vi "UHR-Fleezers Control (host) - Avogadro v3.vi"() -> ()   [LabVIEW 2014] (continued)
                                frame #1 {
                                n2744 = Wait (ms)(milliseconds to wait=u32 500) -> ()  [unwired: 1 out]
                                }
                                frame #2 {
                                n2745 = local read "Shift confocal"() -> (w4245:bool)
                                n2746 = local read "Mean"() -> (w4247:dbl)
                                n2747 = Greater?(x=w4247, y=11.0) -> (0:w4244:bool)
                                n2748 = Not(x=w4244) -> (.not. x?=w4243:bool)
                                n2749 = And(x=w4243, y=w4245) -> (x .and. y?=w4241:bool)
                                n2750 = And(x=w4244, y=w4245) -> (x .and. y?=w4242:bool)
                                n2751 = case shown="True" w4242 {
                                frame False {
                                }
                                frame True {
                                n2752 = local read "Confocal Y 2 (V)"() -> (w4251:dbl)
                                n2753 = local read "Confocal X 2 (V)"() -> (w4250:dbl)
                                n2754 = property on="AO2" class="Slide (strict)"("Val(Sgnl)"=w4250) -> ()  [unwired: 2 in, 2 out]
                                n2755 = property on="AO1" class="Slide (strict)"("Val(Sgnl)"=w4251) -> ()  [unwired: 2 in, 2 out]
                                }
                                }
                                n2756 = case shown="True" w4241 {
                                frame False {
                                }
                                frame True {
                                n2757 = local read "Confocal X 1 (V)"() -> (w4248:dbl)
                                n2758 = local read "Confocal Y 1 (V)"() -> (w4249:dbl)
                                n2759 = property on="AO2" class="Slide (strict)"("Val(Sgnl)"=w4248) -> ()  [unwired: 2 in, 2 out]
                                n2760 = property on="AO1" class="Slide (strict)"("Val(Sgnl)"=w4249) -> ()  [unwired: 2 in, 2 out]
                                }
                                }
                                }
                                }
                                }
                                }
                                }
                                }
                                }
                                frame "Image" {
                                n2761 = property on="Confocal Image" class="Bool (strict)"("Val(Sgnl)"=TRUE ("Value (Signaling)")) -> ()  [unwired: 2 in, 2 out]
                                }
                              }
                              n2762 = local write "Fl. High"(FALSE ("Fl. High")) -> ()
                              n2763 = local read "Time (s)"() -> (w4185:dbl)
                            }
                            frame #1 {
                              n2764 = case shown="True" "Auto F Reset" {
                                tunnel: w4257 -> [_ w4262]
                                tunnel: w4256 -> [_ w4261]
                                tunnel: w4255 -> [_ w4260]
                                tunnel: w4254 -> [_ w4259]
                                frame False {
                                }
                                frame True {
                                n2765 = node-c288() -> (w4264:T43)  [unwired: 4 in]
                                n2766 = timed-loop {
                                timing: w4264 -> [_]
                                timing-out: [_] -> w4263
                                tunnel: w4262 -> [w4269]
                                tunnel: w4261 -> [w4268]
                                tunnel: w4260 -> [w4267]
                                tunnel: w4259 -> [w4266]
                                stop <- w4265 stop-if-true
                                n2767 = node-c288() -> ()  [unwired: 1 in, 1 out]
                                n2768 = local read "Fl. Delta Thresh. (kHz)"() -> (w4278:dbl)
                                n2769 = local read "APD to Watch"() -> (w4279:bool)
                                n2770 = local read "Delta Fl. 1"() -> (w4280:dbl)
                                n2771 = local read "Delta Fl. 2"() -> (w4281:dbl)
                                n2772 = local read "Fl. Triggered..."() -> (w4272:bool)
                                n2773 = local read "Stop All"() -> (w4273:bool)
                                n2774 = local read "Reset Force"() -> (w4271:bool)
                                n2775 = Multiply(x=w4278, y=1000.0) -> (x*y=w4276:dbl)
                                n2776 = Select(t=w4280, s=w4279, f=w4281) -> (s? t:f=w4275:dbl)
                                n2777 = Not(x=w4272) -> (.not. x?=w4270:bool)
                                n2778 = Greater?(x=w4275, y=w4276) -> (0:w4274:bool)
                                n2779 = Compound Arithmetic op=OR(w4274, w4273, w4270, w4271) -> (w4265:bool)
                                n2780 = case shown="True" w4265 {
                                tunnel: w4269 -> [_ w4285]
                                tunnel: w4268 -> [_ w4289]
                                tunnel: w4267 -> [_ w4288]
                                tunnel: w4266 -> [_ w4287]
                                frame False {
                                }
                                frame True {
                                n2781 = case shown="\"Yank\"" w4289 {
                                tunnel: w4288 -> [_ w4299]
                                tunnel: w4287 -> [_ w4297]
                                frame "Image", Default {
                                }
                                frame "Yank" {
                                n2782 = flat-sequence {
                                tunnel: [w4302] -> w4300
                                tunnel: w4299 -> [w4302]
                                tunnel: [w4301] -> w4298
                                tunnel: w4297 -> [w4301]
                                tunnel: w4300 -> [w4308]
                                tunnel: w4298 -> [w4306]
                                frame #0 {
                                n2783 = local read "Yank Delay (s)"() -> (w4305:dbl)
                                n2784 = Multiply(x=w4305, y=1000.0) -> (x*y=w4303:dbl)
                                n2785 = Wait (ms)(milliseconds to wait=w4303) -> ()  [unwired: 1 out]
                                }
                                frame #1 {
                                n2786 = local read "Yank to which?"() -> (w4307:bool)
                                n2787 = case shown="False" w4307 {
                                tunnel: w4308 -> [_ w4336]
                                tunnel: w4306 -> [w4309 _]
                                frame False {
                                n2788 = flat-sequence {
                                tunnel: w4309 -> [w4310]
                                frame #0 {
                                n2789 = property on="Trap Pos FB SP" class="DigNum (strict)"("Val(Sgnl)"=w4310) -> ()  [unwired: 2 in, 2 out]
                                }
                                frame #1 {
                                n2790 = Wait (ms)(milliseconds to wait=u32 700) -> ()  [unwired: 1 out]
                                }
                                frame #2 {
                                n2791 = local read "Action (%)"() -> (w4315:dbl)
                                n2792 = Absolute Value(x=w4315) -> (abs(x)=w4314:dbl)
                                n2793 = Greater?(x=w4314, y=70.0) -> (0:w4312:bool)
                                n2794 = property on="Remove Action Offset" class="Bool (strict)"("Val(Sgnl)"=w4312) -> ()  [unwired: 2 in, 2 out]
                                }
                                frame #3 {
                                n2795 = for {
                                N: 4 -> [_]
                                n2796 = flat-sequence {
                                frame #0 {
                                n2797 = Wait (ms)(milliseconds to wait=u32 500) -> ()  [unwired: 1 out]
                                }
                                frame #1 {
                                n2798 = local read "Action (%)"() -> (w4321:dbl)
                                n2799 = Absolute Value(x=w4321) -> (abs(x)=w4320:dbl)
                                n2800 = Greater?(x=w4320, y=70.0) -> (0:w4318:bool)
                                n2801 = property on="Remove Action Offset" class="Bool (strict)"("Val(Sgnl)"=w4318) -> ()  [unwired: 2 in, 2 out]
                                }
                                }
                                }
                                }
                                frame #4 {
                                n2802 = Wait (ms)(milliseconds to wait=u32 500) -> ()  [unwired: 1 out]
                                }
                                frame #5 {
                                n2803 = local read "Shift confocal"() -> (w4326:bool)
                                n2804 = local read "Mean"() -> (w4329:dbl)
                                n2805 = Greater?(x=w4329, y=11.0) -> (0:w4325:bool)
                                n2806 = Not(x=w4325) -> (.not. x?=w4324:bool)
                                n2807 = And(x=w4325, y=w4326) -> (x .and. y?=w4327:bool)
                                n2808 = And(x=w4324, y=w4326) -> (x .and. y?=w4323:bool)
                                n2809 = case shown="True" w4327 {
                                frame False {
                                }
                                frame True {
                                n2810 = local read "Confocal X 2 (V)"() -> (w4332:dbl)
                                n2811 = local read "Confocal Y 2 (V)"() -> (w4333:dbl)
                                n2812 = property on="AO2" class="Slide (strict)"("Val(Sgnl)"=w4332) -> ()  [unwired: 2 in, 2 out]
                                n2813 = property on="AO1" class="Slide (strict)"("Val(Sgnl)"=w4333) -> ()  [unwired: 2 in, 2 out]
                                }
                                }
                                n2814 = case shown="True" w4323 {
                                frame False {
                                }
                                frame True {
                                n2815 = local read "Confocal Y 1 (V)"() -> (w4331:dbl)
                                n2816 = local read "Confocal X 1 (V)"() -> (w4330:dbl)
                                n2817 = property on="AO1" class="Slide (strict)"("Val(Sgnl)"=w4331) -> ()  [unwired: 2 in, 2 out]
                                n2818 = property on="AO2" class="Slide (strict)"("Val(Sgnl)"=w4330) -> ()  [unwired: 2 in, 2 out]
                                }
                                }
                                }
                                frame #6 {
                                n2819 = Wait (ms)(milliseconds to wait=u32 1500) -> ()  [unwired: 1 out]
                                }
                                frame #7 {
                                n2820 = property on="Rem fb disp offset" class="Bool (strict)"("Val(Sgnl)"=TRUE ("Value (Signaling)")) -> ()  [unwired: 2 in, 2 out]
                                }
                                }
                                }
                                frame True {
                                n2821 = flat-sequence {
                                tunnel: w4336 -> [w4337]
                                frame #0 {
                                n2822 = property on="Trap Delta (MHz)" class="DigNum (strict)"("Val(Sgnl)"=w4337) -> ()  [unwired: 2 in, 2 out]
                                }
                                frame #1 {
                                n2823 = Wait (ms)(milliseconds to wait=u32 500) -> ()  [unwired: 1 out]
                                }
                                frame #2 {
                                n2824 = local read "Shift confocal"() -> (w4343:bool)
                                n2825 = local read "Mean"() -> (w4344:dbl)
                                n2826 = Greater?(x=w4344, y=11.0) -> (0:w4342:bool)
                                n2827 = And(x=w4342, y=w4343) -> (x .and. y?=w4340:bool)
                                n2828 = Not(x=w4342) -> (.not. x?=w4341:bool)
                                n2829 = And(x=w4341, y=w4343) -> (x .and. y?=w4339:bool)
                                n2830 = case shown="True" w4340 {
                                frame False {
                                }
                                frame True {
                                n2831 = local read "Confocal Y 2 (V)"() -> (w4349:dbl)
                                n2832 = local read "Confocal X 2 (V)"() -> (w4348:dbl)
                                n2833 = property on="AO1" class="Slide (strict)"("Val(Sgnl)"=w4349) -> ()  [unwired: 2 in, 2 out]
                                n2834 = property on="AO2" class="Slide (strict)"("Val(Sgnl)"=w4348) -> ()  [unwired: 2 in, 2 out]
                                }
                                }
                                n2835 = case shown="True" w4339 {
                                frame False {
                                }
                                frame True {
                                n2836 = local read "Confocal Y 1 (V)"() -> (w4347:dbl)
                                n2837 = local read "Confocal X 1 (V)"() -> (w4346:dbl)
                                n2838 = property on="AO2" class="Slide (strict)"("Val(Sgnl)"=w4346) -> ()  [unwired: 2 in, 2 out]
                                n2839 = property on="AO1" class="Slide (strict)"("Val(Sgnl)"=w4347) -> ()  [unwired: 2 in, 2 out]
                                }
                                }
                                }
                                }
                                }
                                }
                                }
                                }
                                }
                                }
                                n2840 = local read "Time (s)"() -> (w4284:dbl)
                                n2841 = Subtract(x=w4285, y=w4284) -> (x-y=w4296:dbl)
                                n2842 = Number To Decimal String(number=w4296, width (-)=i16 0) -> (decimal integer string=w4294:string)
                                n2843 = Concatenate Strings(w4294, " s fluorescence event") -> (w4291:string)
                                n2844 = local read "Messages"() -> (w4292:string)
                                n2845 = local write "Duration (s)"(w4296) -> ()
                                n2846 = call "Update messages.vi"("Message to add"=w4291, "Old message string"=w4292) -> ("New message string"=w4290:string)
                                n2847 = local write "Messages"(w4290) -> ()
                                n2848 = call <vilib>:"Beep.vi"() -> ()  [unwired: 12 in]
                                n2849 = local write "Reset Force"(FALSE ("Force Reset")) -> ()
                                n2850 = local write "Fl. High"(TRUE ("Fl. High")) -> ()
                                n2851 = local write "Waiting"(TRUE ("Waiting")) -> ()
                                }
                                }
                                n2852 = node-c288() -> ()  [unwired: 1 in, 1 out]
                                }
                                n2853 = node-c288(w4263) -> ()  [unwired: 1 out]
                                }
                              }
                            }
                          }
                          n2854 = local read "Trap Delta (MHz)"() -> (w4175:dbl)
                          n2855 = local read "Trap Pos FB SP"() -> (w4173:fxp<+/-,16,1>)
                        }
                      }
                    }
                    frame True {
                      n2856 = flat-sequence {
                        tunnel: w4360 -> [w4370]
                        tunnel: [w4370] -> w4364
                        tunnel: w4363 -> [w4369]
                        tunnel: [w4369] -> w4362
                        tunnel: [w4368] -> w4361
                        tunnel: w4359 -> [w4367]
                        tunnel: [w4366] -> w4358
                        tunnel: w4355 -> [w4365]
                        tunnel: [w4365] -> w4354
                        tunnel: w4364 -> [w4440]
                        tunnel: w4362 -> [w4439]
                        tunnel: w4361 -> [w4438]
                        tunnel: w4358 -> [w4437]
                        tunnel: w4354 -> [w4436]
                        tunnel: [w4437] -> w4357
                        frame #0 {
                          n2857 = call <vilib>:"Beep.vi"() -> ()  [unwired: 3 in, 9 out]
                          n2858 = local write "Waiting"(FALSE ("Waiting")) -> ()
                          n2859 = Increment(x=w4367) -> (x+1=w4366:u8)
                          n2860 = case shown="\"Image\"" w4369 {
                            tunnel: w4366 -> [_ _ w4376]
                            frame "Image" {
                              n2861 = property on="Confocal Image" class="Bool (strict)"("Val(Sgnl)"=TRUE ("Value (Signaling)")) -> ()  [unwired: 2 in, 2 out]
                            }
                            frame "Alarm", Default {
                            }
                            frame "Yank" {
                              n2862 = flat-sequence {
                                tunnel: w4376 -> [w4379]
                                tunnel: [w4378] -> w4375
                                tunnel: ["N Array El"] -> w4374
                                tunnel: w4375 -> [w4393]
                                tunnel: w4374 -> [w4389]
                                frame #0 {
                                n2863 = Multiply(x="Yank Delay (s)", y=1000.0) -> (x*y=w4382:dbl)
                                n2864 = Quotient & Remainder(x=w4379, y="N Array El") -> (x-y*floor(x/y)=w4378:u8)  [unwired: 1 out]
                                n2865 = Wait (ms)(milliseconds to wait=w4382) -> ()  [unwired: 1 out]
                                }
                                frame #1 {
                                n2866 = Random Number (0-1)() -> (number: 0 to 1=w4390:dbl)
                                n2867 = Multiply(x=w4389, y=w4390) -> (x*y=w4388:dbl)
                                n2868 = Round Toward -Infinity(1:w4388) -> (0:w4387:dbl)
                                n2869 = Select(t=w4387, s="Random Choice", f=w4393) -> (s? t:f=w4391:dbl)
                                n2870 = Select(t="Yank to Trap Delta (MHz)", s="Yank to which?", f="Yank to SP") -> (s? t:f=w4384:dbl[])
                                n2871 = Index Array(array=w4384, index=w4391) -> (element=w4394:dbl)
                                n2872 = case shown="False" "Yank to which?" {
                                tunnel: w4394 -> [w4395 w4421]
                                frame False {
                                n2873 = flat-sequence {
                                tunnel: w4395 -> [w4396]
                                frame #0 {
                                n2874 = property on="Trap Pos FB SP" class="DigNum (strict)"("Val(Sgnl)"=w4396) -> ()  [unwired: 2 in, 2 out]
                                }
                                frame #1 {
                                n2875 = Wait (ms)(milliseconds to wait=u32 700) -> ()  [unwired: 1 out]
                                }
                                frame #2 {
                                n2876 = local read "Action (%)"() -> (w4401:dbl)
                                n2877 = Absolute Value(x=w4401) -> (abs(x)=w4400:dbl)
                                n2878 = Greater?(x=w4400, y=70.0) -> (0:w4398:bool)
                                n2879 = property on="Remove Action Offset" class="Bool (strict)"("Val(Sgnl)"=w4398) -> ()  [unwired: 2 in, 2 out]
                                }
                                frame #3 {
                                n2880 = for {
                                N: 4 -> [_]
                                n2881 = flat-sequence {
                                frame #0 {
                                n2882 = Wait (ms)(milliseconds to wait=u32 500) -> ()  [unwired: 1 out]
                                }
                                frame #1 {
                                n2883 = local read "Action (%)"() -> (w4407:dbl)
                                n2884 = Absolute Value(x=w4407) -> (abs(x)=w4406:dbl)
                                n2885 = Greater?(x=w4406, y=70.0) -> (0:w4404:bool)
                                n2886 = property on="Remove Action Offset" class="Bool (strict)"("Val(Sgnl)"=w4404) -> ()  [unwired: 2 in, 2 out]
                                }
                                }
                                }
                                }
                                frame #4 {
                                n2887 = local read "Shift confocal"() -> (w4411:bool)
                                n2888 = local read "Mean"() -> (w4414:dbl)
                                n2889 = Greater?(x=w4414, y=11.0) -> (0:w4410:bool)
                                n2890 = Not(x=w4410) -> (.not. x?=w4409:bool)
                                n2891 = And(x=w4409, y=w4411) -> (x .and. y?=w4408:bool)
                                n2892 = And(x=w4410, y=w4411) -> (x .and. y?=w4412:bool)
                                n2893 = case shown="True" w4412 {
                                frame False {
                                }
                                frame True {
                                n2894 = local read "Confocal X 2 (V)"() -> (w4417:dbl)
                                n2895 = local read "Confocal Y 2 (V)"() -> (w4418:dbl)
                                n2896 = property on="AO2" class="Slide (strict)"("Val(Sgnl)"=w4417) -> ()  [unwired: 2 in, 2 out]
                                n2897 = property on="AO1" class="Slide (strict)"("Val(Sgnl)"=w4418) -> ()  [unwired: 2 in, 2 out]
                                }
                                }
                                n2898 = case shown="True" w4408 {
                                frame False {
                                }
                                frame True {
                                n2899 = local read "Confocal X 1 (V)"() -> (w4415:dbl)
                                n2900 = local read "Confocal Y 1 (V)"() -> (w4416:dbl)
                                n2901 = property on="AO1" class="Slide (strict)"("Val(Sgnl)"=w4416) -> ()  [unwired: 2 in, 2 out]
                                n2902 = property on="AO2" class="Slide (strict)"("Val(Sgnl)"=w4415) -> ()  [unwired: 2 in, 2 out]
                                }
                                }
                                }
                                frame #5 {
                                n2903 = Wait (ms)(milliseconds to wait=u32 1500) -> ()  [unwired: 1 out]
                                }
                                frame #6 {
                                n2904 = property on="Rem fb disp offset" class="Bool (strict)"("Val(Sgnl)"=TRUE ("Value (Signaling)")) -> ()  [unwired: 2 in, 2 out]
                                }
                                }
                                }
                                frame True {
                                n2905 = flat-sequence {
                                tunnel: w4421 -> [w4422]
                                frame #0 {
                                n2906 = property on="Trap Delta (MHz)" class="DigNum (strict)"("Val(Sgnl)"=w4422) -> ()  [unwired: 2 in, 2 out]
                                }
                                frame #1 {
                                n2907 = Wait (ms)(milliseconds to wait=u32 500) -> ()  [unwired: 1 out]
                                }
                                frame #2 {
                                n2908 = local read "Shift confocal"() -> (w4426:bool)
                                n2909 = local read "Mean"() -> (w4424:dbl)
                                n2910 = Greater?(x=w4424, y=11.0) -> (0:w4427:bool)
                                n2911 = Not(x=w4427) -> (.not. x?=w4428:bool)
                                n2912 = And(x=w4428, y=w4426) -> (x .and. y?=w4430:bool)
                                n2913 = And(x=w4427, y=w4426) -> (x .and. y?=w4429:bool)
                                n2914 = case shown="True" w4429 {
                                frame False {
                                }
                                frame True {
                                n2915 = local read "Confocal Y 2 (V)"() -> (w4434:dbl)
                                n2916 = local read "Confocal X 2 (V)"() -> (w4433:dbl)
                                n2917 = property on="AO1" class="Slide (strict)"("Val(Sgnl)"=w4434) -> ()  [unwired: 2 in, 2 out]
                                n2918 = property on="AO2" class="Slide (strict)"("Val(Sgnl)"=w4433) -> ()  [unwired: 2 in, 2 out]
                                }
                                }
                                n2919 = case shown="True" w4430 {
                                frame False {
                                }
                                frame True {
                                n2920 = local read "Confocal X 1 (V)"() -> (w4431:dbl)
                                n2921 = local read "Confocal Y 1 (V)"() -> (w4432:dbl)
                                n2922 = property on="AO2" class="Slide (strict)"("Val(Sgnl)"=w4431) -> ()  [unwired: 2 in, 2 out]
                                n2923 = property on="AO1" class="Slide (strict)"("Val(Sgnl)"=w4432) -> ()  [unwired: 2 in, 2 out]
                                }
                                }
                                }
                                }
                                }
                                }
                                }
                              }
                            }
                          }
                          n2924 = local read "Time (s)"() -> (w4368:dbl)
                          "Fl. High" <- TRUE ("Yanking")
                        }
                        frame #1 {
                          n2925 = local read "Auto F Reset"() -> (w4435:bool)
                          n2926 = case shown="True" w4435 {
                            tunnel: w4440 -> [_ w4444]
                            tunnel: w4439 -> [_ w4443]
                            tunnel: w4438 -> [_ w4442]
                            tunnel: w4436 -> [_ w4441]
                            frame False {
                            }
                            frame True {
                              n2927 = node-c288() -> (w4446:T43)  [unwired: 4 out]
                              n2928 = timed-loop {
                                timing: w4446 -> [_]
                                timing-out: [_] -> w4445
                                tunnel: w4444 -> [w4464]
                                tunnel: w4443 -> [w4463]
                                tunnel: w4442 -> [w4462]
                                tunnel: w4441 -> [w4461]
                                stop <- w4447 stop-if-true
                                n2929 = node-c288() -> ()  [unwired: 2 out]
                                n2930 = local read "Fl. Delta Thresh. (kHz)"() -> (w4455:dbl)
                                n2931 = local read "Fl. Triggered..."() -> (w4460:bool)
                                n2932 = local read "Delta Fl. 1"() -> (w4451:dbl)
                                n2933 = local read "Delta Fl. 2"() -> (w4449:dbl)
                                n2934 = local read "Stop All"() -> (w4458:bool)
                                n2935 = local read "APD to Watch"() -> (w4450:bool)
                                n2936 = Select(t=w4451, s=w4450, f=w4449) -> (s? t:f=w4448:dbl)
                                n2937 = Not(x=w4460) -> (.not. x?=w4459:bool)
                                n2938 = Multiply(x=w4455, y=1000.0) -> (x*y=w4454:dbl)
                                n2939 = Negate(x=w4454) -> (-x=w4453:dbl)
                                n2940 = Less?(x=w4448, y=w4453) -> (x < y?=w4457:bool)
                                n2941 = Compound Arithmetic op=OR(w4457, w4458, w4459, "Reset Force") -> (w4447:bool)
                                n2942 = case shown="True" w4447 {
                                tunnel: w4464 -> [_ w4479]
                                tunnel: w4463 -> [_ w4478]
                                tunnel: w4462 -> [_ w4468]
                                tunnel: w4461 -> [_ w4470]
                                frame False {
                                }
                                frame True {
                                n2943 = local read "Time (s)"() -> (w4469:dbl)
                                n2944 = case shown="\"Yank\"" w4478 {
                                tunnel: w4479 -> [_ w4482]
                                tunnel: w4470 -> [_ w4480]
                                frame "Image", Default {
                                }
                                frame "Yank" {
                                n2945 = flat-sequence {
                                tunnel: [w4488] -> w4483
                                tunnel: w4482 -> [w4488]
                                tunnel: [w4484] -> w4481
                                tunnel: w4480 -> [w4484]
                                tunnel: w4483 -> [w4491]
                                tunnel: w4481 -> [w4489]
                                frame #0 {
                                n2946 = local read "Yank Delay (s)"() -> (w4487:dbl)
                                n2947 = Multiply(x=w4487, y=1000.0) -> (x*y=w4485:dbl)
                                n2948 = Wait (ms)(milliseconds to wait=w4485) -> ()  [unwired: 1 out]
                                }
                                frame #1 {
                                n2949 = local read "Yank to which?"() -> (w4490:bool)
                                n2950 = case shown="False" w4490 {
                                tunnel: w4491 -> [_ w4518]
                                tunnel: w4489 -> [w4492 _]
                                frame False {
                                n2951 = flat-sequence {
                                tunnel: w4492 -> [w4493]
                                frame #0 {
                                n2952 = property on="Trap Pos FB SP" class="DigNum (strict)"("Val(Sgnl)"=w4493) -> ()  [unwired: 2 in, 2 out]
                                }
                                frame #1 {
                                n2953 = Wait (ms)(milliseconds to wait=u32 700) -> ()  [unwired: 1 out]
                                }
                                frame #2 {
                                n2954 = local read "Action (%)"() -> (w4498:dbl)
                                n2955 = Absolute Value(x=w4498) -> (abs(x)=w4497:dbl)
                                n2956 = Greater?(x=w4497, y=70.0) -> (0:w4495:bool)
                                n2957 = property on="Remove Action Offset" class="Bool (strict)"("Val(Sgnl)"=w4495) -> ()  [unwired: 2 in, 2 out]
                                }
                                frame #3 {
                                n2958 = for {
                                N: 4 -> [_]
                                n2959 = flat-sequence {
                                frame #0 {
                                n2960 = Wait (ms)(milliseconds to wait=u32 500) -> ()  [unwired: 1 out]
                                }
                                frame #1 {
                                n2961 = local read "Action (%)"() -> (w4504:dbl)
                                n2962 = Absolute Value(x=w4504) -> (abs(x)=w4503:dbl)
                                n2963 = Greater?(x=w4503, y=70.0) -> (0:w4501:bool)
                                n2964 = property on="Remove Action Offset" class="Bool (strict)"("Val(Sgnl)"=w4501) -> ()  [unwired: 2 in, 2 out]
                                }
                                }
                                }
                                }
                                frame #4 {
                                n2965 = local read "Shift confocal"() -> (w4509:bool)
                                n2966 = local read "Mean"() -> (w4511:dbl)
                                n2967 = Greater?(x=w4511, y=11.0) -> (0:w4508:bool)
                                n2968 = Not(x=w4508) -> (.not. x?=w4507:bool)
                                n2969 = And(x=w4508, y=w4509) -> (x .and. y?=w4506:bool)
                                n2970 = And(x=w4507, y=w4509) -> (x .and. y?=w4505:bool)
                                n2971 = case shown="True" w4506 {
                                frame False {
                                }
                                frame True {
                                n2972 = local read "Confocal Y 2 (V)"() -> (w4515:dbl)
                                n2973 = local read "Confocal X 2 (V)"() -> (w4514:dbl)
                                n2974 = property on="AO2" class="Slide (strict)"("Val(Sgnl)"=w4514) -> ()  [unwired: 2 in, 2 out]
                                n2975 = property on="AO1" class="Slide (strict)"("Val(Sgnl)"=w4515) -> ()  [unwired: 2 in, 2 out]
                                }
                                }
                                n2976 = case shown="True" w4505 {
                                frame False {
                                }
                                frame True {
                                n2977 = local read "Confocal X 1 (V)"() -> (w4512:dbl)
                                n2978 = local read "Confocal Y 1 (V)"() -> (w4513:dbl)
                                n2979 = property on="AO1" class="Slide (strict)"("Val(Sgnl)"=w4513) -> ()  [unwired: 2 in, 2 out]
                                n2980 = property on="AO2" class="Slide (strict)"("Val(Sgnl)"=w4512) -> ()  [unwired: 2 in, 2 out]
                                }
                                }
                                }
                                frame #5 {
                                n2981 = Wait (ms)(milliseconds to wait=u32 1500) -> ()  [unwired: 1 out]
                                }
                                frame #6 {
                                n2982 = property on="Rem fb disp offset" class="Bool (strict)"("Val(Sgnl)"=TRUE ("Value (Signaling)")) -> ()  [unwired: 2 in, 2 out]
                                }
                                }
                                }
                                frame True {
                                n2983 = flat-sequence {
                                tunnel: w4518 -> [w4519]
                                frame #0 {
                                n2984 = property on="Trap Delta (MHz)" class="DigNum (strict)"("Val(Sgnl)"=w4519) -> ()  [unwired: 2 in, 2 out]
                                }
                                frame #1 {
                                n2985 = Wait (ms)(milliseconds to wait=u32 500) -> ()  [unwired: 1 out]
                                }
                                frame #2 {
                                n2986 = local read "Shift confocal"() -> (w4525:bool)
                                n2987 = local read "Mean"() -> (w4527:dbl)
                                n2988 = Greater?(x=w4527, y=11.0) -> (0:w4524:bool)
                                n2989 = Not(x=w4524) -> (.not. x?=w4523:bool)
                                n2990 = And(x=w4524, y=w4525) -> (x .and. y?=w4522:bool)
                                n2991 = And(x=w4523, y=w4525) -> (x .and. y?=w4521:bool)
                                n2992 = case shown="True" w4522 {
                                frame False {
                                }
                                frame True {
                                n2993 = local read "Confocal Y 2 (V)"() -> (w4531:dbl)
                                n2994 = local read "Confocal X 2 (V)"() -> (w4530:dbl)
                                n2995 = property on="AO2" class="Slide (strict)"("Val(Sgnl)"=w4530) -> ()  [unwired: 2 in, 2 out]
                                n2996 = property on="AO1" class="Slide (strict)"("Val(Sgnl)"=w4531) -> ()  [unwired: 2 in, 2 out]
                                }
                                }
                                n2997 = case shown="True" w4521 {
                                frame False {
                                }
                                frame True {
                                n2998 = local read "Confocal Y 1 (V)"() -> (w4529:dbl)
                                n2999 = local read "Confocal X 1 (V)"() -> (w4528:dbl)
                                n3000 = property on="AO2" class="Slide (strict)"("Val(Sgnl)"=w4528) -> ()  [unwired: 2 in, 2 out]
                                n3001 = property on="AO1" class="Slide (strict)"("Val(Sgnl)"=w4529) -> ()  [unwired: 2 in, 2 out]
                                }
                                }
                                }
                                }
                                }
                                }
                                }
                                }
                                }
                                }
                                n3002 = local read "Messages"() -> (w4477:string)
                                n3003 = Subtract(x=w4469, y=w4468) -> (x-y=w4475:dbl)
                                "Duration (s)" <- w4475
                                n3004 = Number To Decimal String(number=w4475, width (-)=i16 0) -> (decimal integer string=w4473:string)
                                n3005 = Concatenate Strings(w4473, " s fluorescence event." ("string")) -> (w4471:string)
                                n3006 = call "Update messages.vi"("Message to add"=w4471, "Old message string"=w4477) -> ("New message string"=w4476:string)
                                n3007 = local write "Reset Force"(FALSE ("Reset Force")) -> ()
                                n3008 = local write "Waiting"(TRUE ("Waiting")) -> ()
                                n3009 = local write "Messages"(w4476) -> ()
                                n3010 = local write "Fl. High"(FALSE ("Fl. High")) -> ()
                                n3011 = call <vilib>:"Beep.vi"() -> ()  [unwired: 3 in, 9 out]
                                }
                                }
                                n3012 = node-c288() -> ()  [unwired: 2 out]
                              }
                              n3013 = node-c288(w4445) -> ()  [unwired: 1 out]
                            }
                          }
                        }
                      }
                      n3014 = local read "Trap Delta (MHz)"() -> (w4360:dbl)
                      n3015 = local read "Trap Pos FB SP"() -> (w4355:fxp<+/-,16,1>)
                    }
                  }
                }
                frame #1 {
                  n3016 = local read "Stop All"() -> (w4541:bool)
                  n3017 = local read "Fl. Triggered..."() -> (w4539:bool)
                  n3018 = Not(x=w4539) -> (.not. x?=w4540:bool)
                  n3019 = Or(x=w4540, y=w4541) -> (x .or. y?=w4538:bool)
                }
              }
              n3020 = case shown="True" w4132 {
                frame False {
                }
                frame True {
                  n3021 = local read "Confocal Y 1 (V)"() -> (w4142:dbl)
                  n3022 = local read "Confocal X 1 (V)"() -> (w4141:dbl)
                  n3023 = property on="AO2" class="Slide (strict)"("Val(Sgnl)"=w4141) -> ()  [unwired: 2 in, 2 out]
                  n3024 = property on="AO1" class="Slide (strict)"("Val(Sgnl)"=w4142) -> ()  [unwired: 2 in, 2 out]
                }
              }
              n3025 = case shown="True" w4132 {
                frame False {
                }
                frame True {
                  w4140 = FALSE ("Fl. High")
                  n3026 = local write "Waiting"(w4140) -> ()
                  n3027 = local write "Fl. High"(w4140) -> ()
                }
              }
              n3028 = node-c288() -> ()  [unwired: 2 out]
            }
            n3029 = node-c288(w4130) -> ()  [unwired: 1 out]
          }
        }
      }
      event "Start assembly line": Value Change {
        n3030 = event-data() -> ()  [unwired: 7 out]
        n3031 = case shown="True" "Start assembly line" {
          tunnel: w4547 -> [_ w4548]
          frame False {
          }
          frame True {
            n3032 = flat-sequence {
              tunnel: w4548 -> [w4553]
              tunnel: [w4552] -> w4550
              tunnel: w4550 -> [w4585]
              tunnel: [w4584] -> w4549
              tunnel: w4549 -> [w4587]
              tunnel: w4548 -> [w4606]
              frame #0 {
                w4551 = TRUE ("Value (Signaling)")
                n3033 = property on="Vortran Laser ON" class="Bool (strict)"("Val(Sgnl)"=w4551) -> ()  [unwired: 2 in, 2 out]
                "AL Running" <- w4551
              }
              frame #1 {
                n3034 = node-c288() -> (w4555:T43)  [unwired: 4 in]
                n3035 = timed-loop {
                  timing: w4555 -> [_]
                  timing-out: [_] -> w4554
                  tunnel: w4553 -> [w4563]
                  tunnel: [w4558] -> w4552
                  stop <- w4559 stop-if-true
                  n3036 = node-c288() -> ()  [unwired: 1 in, 1 out]
                  n3037 = local read "APD rates cluster"() -> (w4557:T2)
                  n3038 = Multiply(x="Cy3 Fl.  Thresh. (kHz)", y=1000.0) -> (x*y=w4566:dbl)
                  n3039 = Unbundle By Name(w4557) -> ("APD 1 Rate (Hz)"=w4556:dbl)
                  n3040 = Greater?(x=w4556, y=w4566) -> (0:w4562:bool)
                  n3041 = case shown="True" w4562 {
                    tunnel: w4563 -> [_ w4569]
                    tunnel: [TRUE ("Stage Moving") w4568] -> w4561
                    frame False {
                    }
                    frame True {
                      n3042 = flat-sequence {
                        tunnel: w4569 -> [w4574]
                        tunnel: [w4579] -> w4568
                        frame #0 {
                          n3043 = Multiply(x="AL Delay (s)", y=u32 1000) -> (x*y=w4571:u32)
                          n3044 = Wait (ms)(milliseconds to wait=w4571) -> ()  [unwired: 1 out]
                        }
                        frame #1 {
                          n3045 = property on="Vortran Laser ON" class="Bool (strict)"("Val(Sgnl)"=FALSE ("Value (Signaling)")) -> ()  [unwired: 2 in, 2 out]
                        }
                        frame #2 {
                          # "upper spot"
                          n3046 = local read "Saved Stage Positions"() -> (w4577:dbl[][])
                          n3047 = local write "Stage Moving"(TRUE ("Stage Moving")) -> ()
                          n3048 = call "move to saved stage position.vi"("Stage VISA resource name in"=w4574, "Position"=5, "Saved Stage Positions"=w4577) -> ("error out"=w4575:errorcluster)  [unwired: 1 in, 1 out]
                          n3049 = local write "Stage Control Serial Error"(w4575) -> ()
                        }
                        frame #3 {
                          w4579 = FALSE ("Stage Moving")
                          n3050 = call <vilib>:"Beep.vi"() -> ()  [unwired: 3 in, 9 out]
                          n3051 = local write "Stage Moving"(w4579) -> ()
                        }
                      }
                    }
                  }
                  n3052 = local read "Stop assembly line"() -> (w4558:bool)
                  n3053 = Not(x=w4561) -> (.not. x?=w4560:bool)
                  n3054 = node-c288() -> ()  [unwired: 1 in, 1 out]
                  n3055 = Or(x=w4560, y=w4558) -> (x .or. y?=w4559:bool)
                }
                n3056 = node-c288(w4554) -> ()  [unwired: 1 out]
              }
              frame #2 {
                n3057 = Not(x=w4585) -> (.not. x?=w4584:bool)
                n3058 = case shown="True" w4584 {
                  frame False {
                  }
                  frame True {
                    n3059 = property on="Red Laser ON" class="Bool (strict)"("Val(Sgnl)"=TRUE ("Value (Signaling)")) -> ()  [unwired: 2 in, 2 out]
                  }
                }
              }
              frame #3 {
                n3060 = node-c288() -> (w4589:T43)  [unwired: 4 in]
                n3061 = timed-loop {
                  timing: w4589 -> [_]
                  timing-out: [_] -> w4588
                  tunnel: [w4592] -> _
                  tunnel: w4587 -> [w4592]
                  stop <- "Stop assembly line" stop-if-true
                  n3062 = node-c288() -> ()  [unwired: 1 in, 1 out]
                  n3063 = local read "APD rates cluster"() -> (w4591:T2)
                  n3064 = Multiply(x="Cy5 Fl.  Thresh. (kHz)", y=1000.0) -> (x*y=w4598:dbl)
                  n3065 = Unbundle By Name(w4591) -> ("APD 2 Rate (Hz)"=w4590:dbl)
                  n3066 = Greater?(x=w4590, y=w4598) -> (0:w4595:bool)
                  n3067 = And(x=w4595, y=w4592) -> (x .and. y?=w4593:bool)
                  n3068 = case shown="True" w4593 {
                    frame False {
                    }
                    frame True {
                      n3069 = property on="Vortran Laser ON" class="Bool (strict)"("Val(Sgnl)"=TRUE ("Value (Signaling)")) -> ()  [unwired: 2 in, 2 out]
                    }
                  }
                  n3070 = node-c288() -> ()  [unwired: 1 in, 1 out]
                }
                n3071 = node-c288(w4588) -> ()  [unwired: 1 out]
              }
              frame #4 {
                w4605 = FALSE ("Value (Signaling)")
                # "lower spot"
                n3072 = local read "Saved Stage Positions"() -> (w4609:dbl[][])
                n3073 = property on="Red Laser ON" class="Bool (strict)"("Val(Sgnl)"=w4605) -> ()  [unwired: 2 in, 2 out]
                n3074 = property on="Vortran Laser ON" class="Bool (strict)"("Val(Sgnl)"=w4605) -> ()  [unwired: 2 in, 2 out]
                n3075 = local write "Stage Moving"(TRUE ("Stage Moving")) -> ()
                n3076 = local write "Stop assembly line"(FALSE ("Stop assembly line")) -> ()
                n3077 = call "move to saved stage position.vi"("Stage VISA resource name in"=w4606, "Position"=3, "Saved Stage Positions"=w4609) -> ("error out"=w4608:errorcluster)  [unwired: 1 in, 1 out]
                n3078 = local write "Stage Control Serial Error"(w4608) -> ()
              }
              frame #5 {
                w4611 = FALSE ("Stage Moving")
                n3079 = local write "Stage Moving"(w4611) -> ()
                n3080 = local write "AL Running"(w4611) -> ()
                n3081 = call <vilib>:"Beep.vi"() -> ()  [unwired: 3 in, 9 out]
              }
            }
          }
        }
      }
      event "Stop All": Value Change {
        n3082 = event-data() -> ()  [unwired: 7 out]
        n3083 = local read "Stop All"() -> (w4612:bool)
      }
    }
    n3084 = node-c288() -> ()  [unwired: 2 out]
  }
  n3085 = node-c288(w52) -> ()  [unwired: 1 out]
  n3086 = node-c288(w63) -> ()  [unwired: 1 out]
  n3087 = node-c288(w61) -> ()  [unwired: 1 out]
  n3088 = property on="Saved trap pos" class="WFGraph (strict)"("Visible"=FALSE) -> ()  [unwired: 2 in, 2 out]
  n3089 = property on="Trap Delta Graph" class="WFGraph (strict)"("Visible"=TRUE) -> ()  [unwired: 2 in, 2 out]
  n3090 = disable-structure shown="Disabled" {
    disable-tunnel: w55 -> [w4614 _]
    disable-tunnel: w54 -> [w4613 _]
    frame Disabled {
      n3091 = VISA Close(VISA resource name=w4614, error in (no error)=w4613) -> (error out=w4615:errorcluster)
      n3092 = call <vilib>:"Simple Error Handler.vi"("error in (no error)"=w4615) -> ()  [unwired: 1 in, 8 out]
    }
    frame Enabled {
    }
  }
  n3093 = disable-structure shown="Disabled" {
    disable-tunnel: [w4623 _] -> w20
    disable-tunnel: [w4619 _] -> w19
    disable-tunnel: [w4618 _] -> w18
    disable-tunnel: [w4617 _] -> w17
    disable-tunnel: [w4616 _] -> w16
    frame Disabled {
      # "n samples needed for data"
      n3094 = Unbundle By Name("sound format") -> ("sample rate (S/s)"=w4619:dbl)
      n3095 = call <vilib>:"Sound Output Configure.vi"("number of samples/ch"="number of samples/ch", "sample mode"="sample mode", "sound format"="sound format", "device ID"="device ID") -> ("task ID"=w4623:T61)  [unwired: 6 in, 1 out]
      n3096 = local read "DMA Update Period (s)"() -> (w4620:dbl)
      n3097 = Multiply(x=w4620, y=w4619) -> (x*y=w4618:dbl)
      n3098 = for "Sound time base" {
        N: w4618 -> [_]
        tunnel: [w4627] -> w4621 mode=indexing
        i -> [w4627]
      }
      n3099 = Reciprocal(x=w4619) -> (1/x=w4617:dbl)
      n3100 = Multiply(x=w4621, y=w4617) -> (x*y=w4616:dbl[])
    }
    frame Enabled {
    }
  }
  n3101 = timed-loop "Main data acquisition loop (get data, process data for display, and save data to disk)" {
    tunnel: w15 -> [w4763]
    tunnel: w28 -> [w4762]
    tunnel: [w4950] -> w75
    tunnel: [w4945] -> w74
    timing: w68 -> [_]
    timing-out: [_] -> w67
    tunnel: w46 -> [w4878]
    tunnel: [w4792] -> w21
    tunnel: w20 -> [w4791]
    tunnel: w19 -> [w4789]
    tunnel: w18 -> [w4788]
    tunnel: w17 -> [w4787]
    tunnel: w16 -> [w4786]
    stop <- "Stop All" stop-if-true
    w4706 = 3276.7
    w4835 = "Initialize"
    # "Modified by Ronen 180227: Allows for taking confocal image by moving the piezo trap with a bead inside and using trap 1 (AOM) with very low intensity to measure it"
    # "Cursor control of MCL trap position"
    # "Values for plotting"
    # "List of channels in order (X or Y only):\nT1 X (mV)\nT2 X (mV)\nT1 X (nm)\nT2 X (nm)\nT1 FX (pN)\nT2 FX (pN)\nPosition Difference (nm)\nAPD1\nAPD2\nAPD3"
    # "T2 sum"
    # "T1 sum"
    n3102 = node-c288() -> ()  [unwired: 2 out]
    n3103 = First Call?() -> (First Call?: T/F=w4847:bool)
    n3104 = Or(x="Reset", y=w4847) -> (x .or. y?=w4848:bool)
    n3105 = Or(x="Start AOD Scan", y="Trap Raster Scan") -> (x .or. y?=w4906:bool)
    n3106 = case "Reset data stream (manual reset or at begining of some rastering and imaging)" shown="True" w4848 {
      tunnel: w4763 -> [w5821 w5829]
      tunnel: w4762 -> [w5820 w5828]
      tunnel: [w5821 w5823] -> w4782
      tunnel: [w5820 w5822] -> w4783
      frame False {
      }
      frame True {
        w5826 = TRUE ("AI to FIFO")
        n3107 = call "reset FPGA DMA.vi"("error in"=w5828, "FPGA VI Reference In"=w5829) -> ("error out"=w5824:errorcluster, "FPGA VI Reference Out"=w5825:T41)
        n3108 = local write "Overflow (data lost)"(FALSE ("Overflow (data lost)")) -> ()
        n3109 = xnode "Read/Write Control"("FPGA VI Reference In"=w5825, "error in"=w5824, "AI to FIFO"=w5826, "APD to FIFO"=w5826) -> ("FPGA VI Reference Out"=w5823:T41, "error out"=w5822:errorcluster)
      }
    }
    n3110 = case "Start active calibration (oscillate traps precisely)" shown="True" "Active Cal" {
      tunnel: w4783 -> [w5149 w5157]
      tunnel: w4782 -> [w5148 w5158]
      tunnel: [w5149 w5154] -> w4781
      tunnel: [w5148 w5155] -> w4780
      frame False {
      }
      frame True {
        w5150 = TRUE ("APD to FIFO")
        n3111 = call "reset FPGA DMA.vi"("error in"=w5157, "FPGA VI Reference In"=w5158) -> ("error out"=w5151:errorcluster, "FPGA VI Reference Out"=w5152:T41)
        n3112 = local write "Active Cal"(FALSE ("Active Cal")) -> ()
        n3113 = local write "Save Calibration"(TRUE ("Save Calibration")) -> ()
        n3114 = xnode "Read/Write Control"("FPGA VI Reference In"=w5152, "error in"=w5151, "AI to FIFO"=w5150, "APD to FIFO"=w5150) -> ("FPGA VI Reference Out"=w5155:T41, "error out"=w5154:errorcluster)
      }
    }
    n3115 = case shown="True" "Read Lateness and Rel Phase" {
      tunnel: w4763 -> [w5363 w5396]
      tunnel: w4762 -> [w5364 w5395]
      tunnel: [w5363 w5367] -> w4738
      tunnel: [w5364 w5368] -> w4900
      frame False {
      }
      frame True {
        n3116 = xnode "Read/Write Control"("FPGA VI Reference In"=w5396, "error in"=w5395) -> ("FPGA VI Reference Out"=w5367:T41, "error out"=w5368:errorcluster, "GI Relative phase"=→"Vortran relative phase":i16, "Relative phase"=→"Relative phase (AI1)":i16, "AI Late Counter"=→"Late Counter (AI1)":u8, "GI Late Counter"=→"Vortran Late Counter":u8, "MCL Late Counter"=→"MCL Late Counter":u8, "MCL Relative Phase"=→"Relative Phase (MCL)":i16, "APD Acq Relative Phase"=→"APD Acq Relative Phase":i16, "APD 1 Gate Relative Phase"=→"APD 1 Gate Relative Phase":i16, "APD 2 Gate Relative Phase"=→"APD 2 Gate Relative Phase":i16, "APD Acq Late Counter"=→"APD Acq Late Counter":u8, "APD 1 Gate Late Counter"=→"APD 1 Gate Late Counter":u8, "APD 2 Gate Late Counter"=→"APD 2 Gate Late Counter":u8, "Green FB Relative Phase"=→"Relative phase (Green FB)":i16, "GI Relative phase 2"=→"GI relative phase 2":i16, "GI Late Counter 2"=→"GI Late Counter 2":u8, "Trap Pos FIFO Timeout"=→"Trap Pos FIFO Timeout":u16, "Trap AI FIFO Timeout"=→"Trap AI FIFO Timeout":u16, "RI Late Counter"=→"RI Late Counter":u8, "RI Relative phase"=→"RI relative phase":i16, "Green Late Counter"=→"Green AI Late Counter":u8, "BI Late Counter (AO)"=→"Late Counter (BI AO)":u8, "Blue Late Counter (D)"=→"Late Counter (BI DO)":u8, "BI Relative phase (AO)"=→"Relative phase (BI AO)":i16, "BI Relative phase (D)"=→"Relative phase (BI DO)":i16, "APD 3 Gate Late Counter"=→"APD 3 Gate Late Counter":u8, "APD 3 Gate Relative Phase"=→"APD 3 Gate Relative Phase":i16, "EMCCD Late counter"=→"EMCCD Gate Late Counter":u8, "EMCCD relative phase"=→"EMCCD Gate Relative Phase":i16)
      }
    }
    n3117 = Compound Arithmetic op=OR("Start MCL Scan", "Confocal Image", "Confocal Linescan") -> (w4761:bool)
    n3118 = And(x="Save Data (MCL)", y=w4761) -> (x .and. y?=w4923:bool)
    n3119 = case "Start AOM raster scan" shown="True" w4906 {
      tunnel: w4780 -> [w5680 w5690]
      tunnel: w4781 -> [w5679 w5689]
      tunnel: [w5680 w5683] -> w4926
      tunnel: [w5679 w5682] -> w4925
      frame False {
      }
      frame True {
        n3120 = case shown="True" "Restart DMA? (AOD)" {
          tunnel: [w5719 w5721] -> w5684
          tunnel: [w5718 w5720] -> w5685
          tunnel: w5690 -> [w5719 w5723]
          tunnel: w5689 -> [w5718 w5722]
          frame False {
          }
          frame True {
            n3121 = local write "Overflow (data lost)"(FALSE ("Overflow (data lost)")) -> ()
            n3122 = call "reset FPGA DMA.vi"("error in"=w5722, "FPGA VI Reference In"=w5723) -> ("error out"=w5720:errorcluster, "FPGA VI Reference Out"=w5721:T41)
          }
        }
        n3123 = local write "Trap Raster Scan"(FALSE ("Trap Raster Scan")) -> ()
        n3124 = case shown="False" "Move MCL Also?" {
          tunnel: w5685 -> [w5693 w5713]
          tunnel: w5684 -> [w5694 w5714]
          tunnel: [w5692 w5717] -> w5683
          tunnel: [w5691 w5716] -> w5682
          frame False {
            w5695 = TRUE ("AI to FIFO")
            n3125 = xnode "Read/Write Control"("FPGA VI Reference In"=w5694, "error in"=w5693, "AI to FIFO"=w5695, "APD to FIFO"=w5695, "Start scan"=w5695) -> ("FPGA VI Reference Out"=w5692:T41, "error out"=w5691:errorcluster)
          }
          frame True {
            w5711 = FALSE ("1D or 2D Scan?")
            w5715 = TRUE ("AI to FIFO")
            n3126 = local read "Scan Range (nm)"() -> (w5708:dbl)
            n3127 = local read "Scan steps (AOD)"() -> (w5702:u64)
            n3128 = local read "Total Counts (ticks)"() -> (w5703:u16)
            n3129 = local read "Cycles/step (AOD)"() -> (w5701:u64)
            n3130 = local read "Number of F/B Scans (AOD)"() -> (w5710:u16)
            n3131 = Bundle("Scan Range (nm)"=w5708, "MCL Step Position Ratio"="MCL Step Position Ratio", "MCL/AOM Scale Tweak"="MCL/AOM Scale Tweak", "MCL X Cal (nm/V)"="MCL X Cal (nm/V)", "MCL Step Increment (V_int)"="MCL Step Increment (V_int)", "Total Counts (ticks)"=w5703, "Scan steps (AOD)"=w5702, "Cycles/step (AOD)"=w5701) -> (w5700:T66)  [unwired: 1 in]